vi "FlexMag - 23-03-2023.vi"() -> ()   [LabVIEW 2018] (continued)
            n3079 = In Range and Coerce(upper limit=3.0, x=w4898, lower limit=0.0 ("Elapsed Time (s)")) -> (In Range?=w4892:bool)  [unwired: 1 out]
            n3080 = Not(x=w4895) -> (.not. x?=w4894:bool)
            n3081 = local write "ch3 ch vbv timer"(w4894) -> ()
            n3082 = property on="chvbv3 timer tab" class="TabCtl (strict)"("Visible"=w4892) -> ()  [unwired: 2 in, 2 out]
          }
        }
        n3083 = feedback-in #98(w4536) -> ()
        n3084 = case shown="True" w4546 {
          tunnel: [TRUE FALSE] -> w4545
          tunnel: w4544 -> [_ w4913]
          frame False {
          }
          frame True {
            n3085 = call "Elapsed Time17"("Auto Reset"=w4913) -> ("Elapsed Time (s)"=w4918:dbl)  [unwired: 11 in, 7 out]
            n3086 = Greater?(x=w4918, y=3.0) -> (0:w4915:bool)
            n3087 = In Range and Coerce(upper limit=3.0, x=w4918, lower limit=0.0 ("Elapsed Time (s)")) -> (In Range?=w4912:bool)  [unwired: 1 out]
            n3088 = Not(x=w4915) -> (.not. x?=w4914:bool)
            n3089 = local write "ch1 ch vbv timer"(w4914) -> ()
            n3090 = property on="chvbv1 timer tab" class="TabCtl (strict)"("Visible"=w4912) -> ()  [unwired: 2 in, 2 out]
          }
        }
        n3091 = feedback-in #99(w4545) -> ()
        n3092 = case shown="True" w4564 {
          tunnel: [TRUE FALSE] -> w4563
          tunnel: w4562 -> [_ w4959]
          frame False {
          }
          frame True {
            n3093 = call "Elapsed Time12"("Auto Reset"=w4959) -> ("Elapsed Time (s)"=w4964:dbl)  [unwired: 11 in, 7 out]
            n3094 = Greater?(x=w4964, y=3.0) -> (0:w4961:bool)
            n3095 = In Range and Coerce(upper limit=3.0, x=w4964, lower limit=0.0 ("Elapsed Time (s)")) -> (In Range?=w4958:bool)  [unwired: 1 out]
            n3096 = Not(x=w4961) -> (.not. x?=w4960:bool)
            n3097 = local write "ch4 tp bv timer"(w4960) -> ()
            n3098 = property on="tpbv4 timer tab" class="TabCtl (strict)"("Visible"=w4958) -> ()  [unwired: 2 in, 2 out]
          }
        }
        n3099 = feedback-in #100(w4563) -> ()
        n3100 = case shown="True" w4565 {
          tunnel: [TRUE FALSE] -> w4566
          tunnel: w4567 -> [_ w4979]
          frame False {
          }
          frame True {
            n3101 = call "Elapsed Time10"("Auto Reset"=w4979) -> ("Elapsed Time (s)"=w4984:dbl)  [unwired: 11 in, 7 out]
            n3102 = Greater?(x=w4984, y=3.0) -> (0:w4981:bool)
            n3103 = In Range and Coerce(upper limit=3.0, x=w4984, lower limit=0.0 ("Elapsed Time (s)")) -> (In Range?=w4978:bool)  [unwired: 1 out]
            n3104 = Not(x=w4981) -> (.not. x?=w4980:bool)
            n3105 = local write "ch2 tp bv timer"(w4980) -> ()
            n3106 = property on="tpbv2 timer tab" class="TabCtl (strict)"("Visible"=w4978) -> ()  [unwired: 2 in, 2 out]
          }
        }
        n3107 = feedback-in #101(w4566) -> ()
        n3108 = case shown="True" w4559 {
          tunnel: [TRUE FALSE] -> w4560
          tunnel: w4561 -> [_ w4969]
          frame False {
          }
          frame True {
            n3109 = call "Elapsed Time11"("Auto Reset"=w4969) -> ("Elapsed Time (s)"=w4974:dbl)  [unwired: 11 in, 7 out]
            n3110 = Greater?(x=w4974, y=3.0) -> (0:w4971:bool)
            n3111 = In Range and Coerce(upper limit=3.0, x=w4974, lower limit=0.0 ("Elapsed Time (s)")) -> (In Range?=w4968:bool)  [unwired: 1 out]
            n3112 = Not(x=w4971) -> (.not. x?=w4970:bool)
            n3113 = local write "ch3 tp bv timer"(w4970) -> ()
            n3114 = property on="tpbv3 timer tab" class="TabCtl (strict)"("Visible"=w4968) -> ()  [unwired: 2 in, 2 out]
          }
        }
        n3115 = feedback-in #102(w4560) -> ()
        n3116 = case shown="True" w4588 {
          tunnel: [TRUE FALSE] -> w4587
          tunnel: w4586 -> [_ w5039]
          frame False {
          }
          frame True {
            n3117 = call "Elapsed Time4"("Auto Reset"=w5039) -> ("Elapsed Time (s)"=w5044:dbl)  [unwired: 11 in, 7 out]
            n3118 = Greater?(x=w5044, y=3.0) -> (0:w5041:bool)
            n3119 = In Range and Coerce(upper limit=3.0, x=w5044, lower limit=0.0 ("Elapsed Time (s)")) -> (In Range?=w5038:bool)  [unwired: 1 out]
            n3120 = Not(x=w5041) -> (.not. x?=w5040:bool)
            n3121 = property on="mp4 timer tab" class="TabCtl (strict)"("Visible"=w5038) -> ()  [unwired: 2 in, 2 out]
            n3122 = local write "ch4 mp timer"(w5040) -> ()
          }
        }
        n3123 = feedback-in #103(w4587) -> ()
        n3124 = case shown="True" w4570 {
          tunnel: [TRUE FALSE] -> w4569
          tunnel: w4568 -> [_ w4989]
          frame False {
          }
          frame True {
            n3125 = call "Elapsed Time9"("Auto Reset"=w4989) -> ("Elapsed Time (s)"=w4994:dbl)  [unwired: 11 in, 7 out]
            n3126 = Greater?(x=w4994, y=3.0) -> (0:w4991:bool)
            n3127 = In Range and Coerce(upper limit=3.0, x=w4994, lower limit=0.0 ("Elapsed Time (s)")) -> (In Range?=w4988:bool)  [unwired: 1 out]
            n3128 = Not(x=w4991) -> (.not. x?=w4990:bool)
            n3129 = local write "ch1 tp bv timer"(w4990) -> ()
            n3130 = property on="tpbv1 timer tab" class="TabCtl (strict)"("Visible"=w4988) -> ()  [unwired: 2 in, 2 out]
          }
        }
        n3131 = feedback-in #104(w4569) -> ()
        n3132 = case shown="True" w4589 {
          tunnel: [TRUE FALSE] -> w4590
          tunnel: w4591 -> [_ w5059]
          frame False {
          }
          frame True {
            n3133 = call "Elapsed Time2"("Auto Reset"=w5059) -> ("Elapsed Time (s)"=w5064:dbl)  [unwired: 11 in, 7 out]
            n3134 = Greater?(x=w5064, y=3.0) -> (0:w5061:bool)
            n3135 = In Range and Coerce(upper limit=3.0, x=w5064, lower limit=0.0 ("Elapsed Time (s)")) -> (In Range?=w5058:bool)  [unwired: 1 out]
            n3136 = Not(x=w5061) -> (.not. x?=w5060:bool)
            n3137 = property on="mp2 timer tab" class="TabCtl (strict)"("Visible"=w5058) -> ()  [unwired: 2 in, 2 out]
            n3138 = local write "ch2 mp timer"(w5060) -> ()
          }
        }
        n3139 = feedback-in #105(w4590) -> ()
        n3140 = case shown="True" w4583 {
          tunnel: [TRUE FALSE] -> w4584
          tunnel: w4585 -> [_ w5049]
          frame False {
          }
          frame True {
            n3141 = call "Elapsed Time3"("Auto Reset"=w5049) -> ("Elapsed Time (s)"=w5054:dbl)  [unwired: 11 in, 7 out]
            n3142 = Greater?(x=w5054, y=3.0) -> (0:w5051:bool)
            n3143 = In Range and Coerce(upper limit=3.0, x=w5054, lower limit=0.0 ("Elapsed Time (s)")) -> (In Range?=w5048:bool)  [unwired: 1 out]
            n3144 = Not(x=w5051) -> (.not. x?=w5050:bool)
            n3145 = property on="mp3 timer tab" class="TabCtl (strict)"("Visible"=w5048) -> ()  [unwired: 2 in, 2 out]
            n3146 = local write "ch3 mp timer"(w5050) -> ()
          }
        }
        n3147 = feedback-in #106(w4584) -> ()
        n3148 = case shown="True" w4594 {
          tunnel: [TRUE FALSE] -> w4593
          tunnel: w4592 -> [_ w5068]
          frame False {
          }
          frame True {
            n3149 = call "Elapsed Time"("Auto Reset"=w5068) -> ("Elapsed Time (s)"=w5074:dbl)  [unwired: 11 in, 7 out]
            n3150 = Greater?(x=w5074, y=3.0) -> (0:w5070:bool)
            n3151 = In Range and Coerce(upper limit=3.0, x=w5074, lower limit=0.0 ("Elapsed Time (s)")) -> (In Range?=w5071:bool)  [unwired: 1 out]
            n3152 = Not(x=w5070) -> (.not. x?=w5069:bool)
            n3153 = property on="mp1 timer tab" class="TabCtl (strict)"("Visible"=w5071) -> ()  [unwired: 2 in, 2 out]
            n3154 = local write "ch1 mp timer"(w5069) -> ()
          }
        }
        n3155 = feedback-in #107(w4593) -> ()
        n3156 = local read "ch4 pc gv timer"() -> (w4529:bool)
        n3157 = local read "ch2 pc gv timer"() -> (w4528:bool)
        n3158 = local read "ch3 pc gv timer"() -> (w4534:bool)
        n3159 = local read "ch1 pc gv timer"() -> (w4523:bool)
        n3160 = local read "ch4 pl vbv timer"() -> (w4577:bool)
        n3161 = local read "ch4 tp timer"() -> (w4481:bool)
        n3162 = local read "ch1 pl vbv timer"() -> (w4571:bool)
        n3163 = local read "ch2 pl vbv timer"() -> (w4576:bool)
        n3164 = local read "ch3 pl vbv timer"() -> (w4582:bool)
        n3165 = local read "ch2 tp timer"() -> (w4480:bool)
        n3166 = local read "ch3 tp timer"() -> (w4486:bool)
        n3167 = local read "ch1 tp timer"() -> (w4475:bool)
        n3168 = local read "ch4 cc timer"() -> (w4505:bool)
        n3169 = local read "ch2 cc timer"() -> (w4504:bool)
        n3170 = local read "ch3 cc timer"() -> (w4510:bool)
        n3171 = local read "ch1 cc timer"() -> (w4499:bool)
        n3172 = local read "ch4 tp timer"() -> (w4553:bool)
        n3173 = local read "ch2 tp timer"() -> (w4552:bool)
        n3174 = local read "ch3 tp timer"() -> (w4558:bool)
        n3175 = local read "ch1 tp timer"() -> (w4547:bool)
        n3176 = feedback #108() -> (w4483:bool)  [unwired: 1 in]
        n3177 = feedback #109() -> (w4478:bool)  [unwired: 1 in]
        n3178 = feedback #110() -> (w4484:bool)  [unwired: 1 in]
        n3179 = feedback #111() -> (w4477:bool)  [unwired: 1 in]
        n3180 = feedback #112() -> (w4507:bool)  [unwired: 1 in]
        n3181 = feedback #113() -> (w4531:bool)  [unwired: 1 in]
        n3182 = feedback #114() -> (w4502:bool)  [unwired: 1 in]
        n3183 = feedback #115() -> (w4508:bool)  [unwired: 1 in]
        n3184 = feedback #116() -> (w4526:bool)  [unwired: 1 in]
        n3185 = feedback #117() -> (w4532:bool)  [unwired: 1 in]
        n3186 = feedback #118() -> (w4501:bool)  [unwired: 1 in]
        n3187 = feedback #119() -> (w4525:bool)  [unwired: 1 in]
        n3188 = feedback #120() -> (w4555:bool)  [unwired: 1 in]
        n3189 = feedback #121() -> (w4550:bool)  [unwired: 1 in]
        n3190 = feedback #122() -> (w4556:bool)  [unwired: 1 in]
        n3191 = feedback #123() -> (w4549:bool)  [unwired: 1 in]
        n3192 = feedback #124() -> (w4579:bool)  [unwired: 1 in]
        n3193 = feedback #125() -> (w4573:bool)  [unwired: 1 in]
        n3194 = feedback #126() -> (w4574:bool)  [unwired: 1 in]
        n3195 = feedback #127() -> (w4580:bool)  [unwired: 1 in]
        n3196 = local read "ch4 trnsbp right timer"() -> (w4462:bool)
        n3197 = local read "ch2 trnsbp right timer"() -> (w4469:bool)
        n3198 = local read "ch3 trnsbp right timer"() -> (w4468:bool)
        n3199 = local read "ch2 trnsbp left timer"() -> (w4463:bool)
        n3200 = local read "ch3 trnsbp left timer"() -> (w4457:bool)
        n3201 = local read "ch1 trnsbp left timer"() -> (w4474:bool)
        n3202 = case shown="True" w4481 {
          tunnel: [TRUE FALSE] -> w4482
          tunnel: w4483 -> [_ w4687]
          frame False {
          }
          frame True {
            n3203 = call "Elapsed Time44"("Auto Reset"=w4687) -> ("Elapsed Time (s)"=w4692:dbl)  [unwired: 11 in, 7 out]
            n3204 = Greater?(x=w4692, y=3.0) -> (0:w4689:bool)
            n3205 = In Range and Coerce(upper limit=3.0, x=w4692, lower limit=0.0 ("Elapsed Time (s)")) -> (In Range?=w4686:bool)  [unwired: 1 out]
            n3206 = Not(x=w4689) -> (.not. x?=w4688:bool)
            n3207 = property on="tp4 timer tab" class="TabCtl (strict)"("Visible"=w4686) -> ()  [unwired: 2 in, 2 out]
            n3208 = local write "ch4 tp timer"(w4688) -> ()
          }
        }
        n3209 = feedback-in #108(w4482) -> ()
        n3210 = case shown="True" w4480 {
          tunnel: [TRUE FALSE] -> w4479
          tunnel: w4478 -> [_ w4707]
          frame False {
          }
          frame True {
            n3211 = call "Elapsed Time42"("Auto Reset"=w4707) -> ("Elapsed Time (s)"=w4712:dbl)  [unwired: 11 in, 7 out]
            n3212 = Greater?(x=w4712, y=3.0) -> (0:w4709:bool)
            n3213 = In Range and Coerce(upper limit=3.0, x=w4712, lower limit=0.0 ("Elapsed Time (s)")) -> (In Range?=w4706:bool)  [unwired: 1 out]
            n3214 = Not(x=w4709) -> (.not. x?=w4708:bool)
            n3215 = property on="tp2 timer tab" class="TabCtl (strict)"("Visible"=w4706) -> ()  [unwired: 2 in, 2 out]
            n3216 = local write "ch2 tp timer"(w4708) -> ()
          }
        }
        n3217 = feedback-in #109(w4479) -> ()
        n3218 = case shown="True" w4486 {
          tunnel: [TRUE FALSE] -> w4485
          tunnel: w4484 -> [_ w4697]
          frame False {
          }
          frame True {
            n3219 = call "Elapsed Time43"("Auto Reset"=w4697) -> ("Elapsed Time (s)"=w4702:dbl)  [unwired: 11 in, 7 out]
            n3220 = Greater?(x=w4702, y=3.0) -> (0:w4699:bool)
            n3221 = In Range and Coerce(upper limit=3.0, x=w4702, lower limit=0.0 ("Elapsed Time (s)")) -> (In Range?=w4696:bool)  [unwired: 1 out]
            n3222 = Not(x=w4699) -> (.not. x?=w4698:bool)
            n3223 = property on="tp3 timer tab" class="TabCtl (strict)"("Visible"=w4696) -> ()  [unwired: 2 in, 2 out]
            n3224 = local write "ch3 tp timer"(w4698) -> ()
          }
        }
        n3225 = feedback-in #110(w4485) -> ()
        n3226 = case shown="True" w4475 {
          tunnel: [TRUE FALSE] -> w4476
          tunnel: w4477 -> [_ w4717]
          frame False {
          }
          frame True {
            n3227 = call "Elapsed Time41"("Auto Reset"=w4717) -> ("Elapsed Time (s)"=w4722:dbl)  [unwired: 11 in, 7 out]
            n3228 = Greater?(x=w4722, y=3.0) -> (0:w4719:bool)
            n3229 = In Range and Coerce(upper limit=3.0, x=w4722, lower limit=0.0 ("Elapsed Time (s)")) -> (In Range?=w4716:bool)  [unwired: 1 out]
            n3230 = Not(x=w4719) -> (.not. x?=w4718:bool)
            n3231 = property on="tp1 timer tab" class="TabCtl (strict)"("Visible"=w4716) -> ()  [unwired: 2 in, 2 out]
            n3232 = local write "ch1 tp timer"(w4718) -> ()
          }
        }
        n3233 = feedback-in #111(w4476) -> ()
        n3234 = case shown="True" w4505 {
          tunnel: [TRUE FALSE] -> w4506
          tunnel: w4507 -> [_ w4767]
          frame False {
          }
          frame True {
            n3235 = call "Elapsed Time32"("Auto Reset"=w4767) -> ("Elapsed Time (s)"=w4772:dbl)  [unwired: 11 in, 7 out]
            n3236 = Greater?(x=w4772, y=3.0) -> (0:w4769:bool)
            n3237 = In Range and Coerce(upper limit=3.0, x=w4772, lower limit=0.0 ("Elapsed Time (s)")) -> (In Range?=w4766:bool)  [unwired: 1 out]
            n3238 = Not(x=w4769) -> (.not. x?=w4768:bool)
            n3239 = local write "ch4 cc timer"(w4768) -> ()
            n3240 = property on="cc4 timer tab" class="TabCtl (strict)"("Visible"=w4766) -> ()  [unwired: 2 in, 2 out]
          }
        }
        n3241 = feedback-in #112(w4506) -> ()
        n3242 = case shown="True" w4529 {
          tunnel: [TRUE FALSE] -> w4530
          tunnel: w4531 -> [_ w4846]
          frame False {
          }
          frame True {
            n3243 = call "Elapsed Time24"("Auto Reset"=w4846) -> ("Elapsed Time (s)"=w4851:dbl)  [unwired: 11 in, 7 out]
            n3244 = Greater?(x=w4851, y=3.0) -> (0:w4848:bool)
            n3245 = In Range and Coerce(upper limit=3.0, x=w4851, lower limit=0.0 ("Elapsed Time (s)")) -> ()  [unwired: 2 out]
            n3246 = Not(x=w4848) -> (.not. x?=w4847:bool)
            n3247 = local write "ch4 pc gv timer"(w4847) -> ()
          }
        }
        n3248 = feedback-in #113(w4530) -> ()
        n3249 = case shown="True" w4504 {
          tunnel: [TRUE FALSE] -> w4503
          tunnel: w4502 -> [_ w4787]
          frame False {
          }
          frame True {
            n3250 = call "Elapsed Time30"("Auto Reset"=w4787) -> ("Elapsed Time (s)"=w4792:dbl)  [unwired: 11 in, 7 out]
            n3251 = Greater?(x=w4792, y=3.0) -> (0:w4789:bool)
            n3252 = In Range and Coerce(upper limit=3.0, x=w4792, lower limit=0.0 ("Elapsed Time (s)")) -> (In Range?=w4786:bool)  [unwired: 1 out]
            n3253 = Not(x=w4789) -> (.not. x?=w4788:bool)
            n3254 = property on="cc2 timer tab" class="TabCtl (strict)"("Visible"=w4786) -> ()  [unwired: 2 in, 2 out]
            n3255 = local write "ch2 cc timer"(w4788) -> ()
          }
        }
        n3256 = feedback-in #114(w4503) -> ()
        n3257 = case shown="True" w4510 {
          tunnel: [TRUE FALSE] -> w4509
          tunnel: w4508 -> [_ w4777]
          frame False {
          }
          frame True {
            n3258 = call "Elapsed Time31"("Auto Reset"=w4777) -> ("Elapsed Time (s)"=w4782:dbl)  [unwired: 11 in, 7 out]
            n3259 = Greater?(x=w4782, y=3.0) -> (0:w4779:bool)
            n3260 = In Range and Coerce(upper limit=3.0, x=w4782, lower limit=0.0 ("Elapsed Time (s)")) -> (In Range?=w4776:bool)  [unwired: 1 out]
            n3261 = Not(x=w4779) -> (.not. x?=w4778:bool)
            n3262 = local write "ch3 cc timer"(w4778) -> ()
            n3263 = property on="cc3 timer tab" class="TabCtl (strict)"("Visible"=w4776) -> ()  [unwired: 2 in, 2 out]
          }
        }
        n3264 = feedback-in #115(w4509) -> ()
        n3265 = case shown="True" w4528 {
          tunnel: [TRUE FALSE] -> w4527
          tunnel: w4526 -> [_ w4864]
          frame False {
          }
          frame True {
            n3266 = call "Elapsed Time22"("Auto Reset"=w4864) -> ("Elapsed Time (s)"=w4869:dbl)  [unwired: 11 in, 7 out]
            n3267 = Greater?(x=w4869, y=3.0) -> (0:w4866:bool)
            n3268 = In Range and Coerce(upper limit=3.0, x=w4869, lower limit=0.0 ("Elapsed Time (s)")) -> ()  [unwired: 2 out]
            n3269 = Not(x=w4866) -> (.not. x?=w4865:bool)
            n3270 = local write "ch2 pc gv timer"(w4865) -> ()
          }
        }
        n3271 = feedback-in #116(w4527) -> ()
        n3272 = case shown="True" w4534 {
          tunnel: [TRUE FALSE] -> w4533
          tunnel: w4532 -> [_ w4855]
          frame False {
          }
          frame True {
            n3273 = call "Elapsed Time23"("Auto Reset"=w4855) -> ("Elapsed Time (s)"=w4860:dbl)  [unwired: 11 in, 7 out]
            n3274 = Greater?(x=w4860, y=3.0) -> (0:w4857:bool)
            n3275 = In Range and Coerce(upper limit=3.0, x=w4860, lower limit=0.0 ("Elapsed Time (s)")) -> ()  [unwired: 2 out]
            n3276 = Not(x=w4857) -> (.not. x?=w4856:bool)
            n3277 = local write "ch3 pc gv timer"(w4856) -> ()
          }
        }
        n3278 = feedback-in #117(w4533) -> ()
        n3279 = case shown="True" w4499 {
          tunnel: [TRUE FALSE] -> w4500
          tunnel: w4501 -> [_ w4797]
          frame False {
          }
          frame True {
            n3280 = call "Elapsed Time29"("Auto Reset"=w4797) -> ("Elapsed Time (s)"=w4802:dbl)  [unwired: 11 in, 7 out]
            n3281 = Greater?(x=w4802, y=3.0) -> (0:w4799:bool)
            n3282 = In Range and Coerce(upper limit=3.0, x=w4802, lower limit=0.0 ("Elapsed Time (s)")) -> (In Range?=w4796:bool)  [unwired: 1 out]
            n3283 = Not(x=w4799) -> (.not. x?=w4798:bool)
            n3284 = local write "ch1 cc timer"(w4798) -> ()
            n3285 = property on="cc1 timer tab" class="TabCtl (strict)"("Visible"=w4796) -> ()  [unwired: 2 in, 2 out]
          }
        }
        n3286 = feedback-in #118(w4500) -> ()
        n3287 = case shown="True" w4523 {
          tunnel: [TRUE FALSE] -> w4524
          tunnel: w4525 -> [_ w4873]
          frame False {
          }
          frame True {
            n3288 = call "Elapsed Time21"("Auto Reset"=w4873) -> ("Elapsed Time (s)"=w4878:dbl)  [unwired: 11 in, 7 out]
            n3289 = Greater?(x=w4878, y=3.0) -> (0:w4875:bool)
            n3290 = In Range and Coerce(upper limit=3.0, x=w4878, lower limit=0.0 ("Elapsed Time (s)")) -> ()  [unwired: 2 out]
            n3291 = Not(x=w4875) -> (.not. x?=w4874:bool)
            n3292 = local write "ch1 pc gv timer"(w4874) -> ()
          }
        }
        n3293 = feedback-in #119(w4524) -> ()
        n3294 = case shown="True" w4553 {
          tunnel: [TRUE FALSE] -> w4554
          tunnel: w4555 -> [_ w4922]
          frame False {
          }
          frame True {
            n3295 = call "Elapsed Time16"("Auto Reset"=w4922) -> ("Elapsed Time (s)"=w4927:dbl)  [unwired: 11 in, 7 out]
            n3296 = Greater?(x=w4927, y=3.0) -> (0:w4924:bool)
            n3297 = In Range and Coerce(upper limit=3.0, x=w4927, lower limit=0.0 ("Elapsed Time (s)")) -> ()  [unwired: 2 out]
            n3298 = Not(x=w4924) -> (.not. x?=w4923:bool)
            n3299 = local write "ch4 tp timer"(w4923) -> ()
          }
        }
        n3300 = feedback-in #120(w4554) -> ()
        n3301 = case shown="True" w4552 {
          tunnel: [TRUE FALSE] -> w4551
          tunnel: w4550 -> [_ w4940]
          frame False {
          }
          frame True {
            n3302 = call "Elapsed Time14"("Auto Reset"=w4940) -> ("Elapsed Time (s)"=w4945:dbl)  [unwired: 11 in, 7 out]
            n3303 = Greater?(x=w4945, y=3.0) -> (0:w4942:bool)
            n3304 = In Range and Coerce(upper limit=3.0, x=w4945, lower limit=0.0 ("Elapsed Time (s)")) -> ()  [unwired: 2 out]
            n3305 = Not(x=w4942) -> (.not. x?=w4941:bool)
            n3306 = local write "ch2 tp timer"(w4941) -> ()
          }
        }
        n3307 = feedback-in #121(w4551) -> ()
        n3308 = case shown="True" w4558 {
          tunnel: [TRUE FALSE] -> w4557
          tunnel: w4556 -> [_ w4931]
          frame False {
          }
          frame True {
            n3309 = call "Elapsed Time15"("Auto Reset"=w4931) -> ("Elapsed Time (s)"=w4936:dbl)  [unwired: 11 in, 7 out]
            n3310 = Greater?(x=w4936, y=3.0) -> (0:w4933:bool)
            n3311 = In Range and Coerce(upper limit=3.0, x=w4936, lower limit=0.0 ("Elapsed Time (s)")) -> ()  [unwired: 2 out]
            n3312 = Not(x=w4933) -> (.not. x?=w4932:bool)
            n3313 = local write "ch3 tp timer"(w4932) -> ()
          }
        }
        n3314 = feedback-in #122(w4557) -> ()
        n3315 = case shown="True" w4547 {
          tunnel: [TRUE FALSE] -> w4548
          tunnel: w4549 -> [_ w4949]
          frame False {
          }
          frame True {
            n3316 = call "Elapsed Time13"("Auto Reset"=w4949) -> ("Elapsed Time (s)"=w4954:dbl)  [unwired: 11 in, 7 out]
            n3317 = Greater?(x=w4954, y=3.0) -> (0:w4951:bool)
            n3318 = In Range and Coerce(upper limit=3.0, x=w4954, lower limit=0.0 ("Elapsed Time (s)")) -> ()  [unwired: 2 out]
            n3319 = Not(x=w4951) -> (.not. x?=w4950:bool)
            n3320 = local write "ch1 tp timer"(w4950) -> ()
          }
        }
        n3321 = feedback-in #123(w4548) -> ()
        n3322 = case shown="True" w4577 {
          tunnel: [TRUE FALSE] -> w4578
          tunnel: w4579 -> [_ w4999]
          frame False {
          }
          frame True {
            n3323 = call "Elapsed Time8"("Auto Reset"=w4999) -> ("Elapsed Time (s)"=w5004:dbl)  [unwired: 11 in, 7 out]
            n3324 = Greater?(x=w5004, y=3.0) -> (0:w5001:bool)
            n3325 = In Range and Coerce(upper limit=3.0, x=w5004, lower limit=0.0 ("Elapsed Time (s)")) -> (In Range?=w4998:bool)  [unwired: 1 out]
            n3326 = Not(x=w5001) -> (.not. x?=w5000:bool)
            n3327 = local write "ch4 pl vbv timer"(w5000) -> ()
            n3328 = property on="plvbv4 timer tab" class="TabCtl (strict)"("Visible"=w4998) -> ()  [unwired: 2 in, 2 out]
          }
        }
        n3329 = feedback-in #124(w4578) -> ()
        n3330 = case shown="True" w4571 {
          tunnel: [TRUE FALSE] -> w4572
          tunnel: w4573 -> [_ w5029]
          frame False {
          }
          frame True {
            n3331 = call "Elapsed Time5"("Auto Reset"=w5029) -> ("Elapsed Time (s)"=w5034:dbl)  [unwired: 11 in, 7 out]
            n3332 = Greater?(x=w5034, y=3.0) -> (0:w5031:bool)
            n3333 = In Range and Coerce(upper limit=3.0, x=w5034, lower limit=0.0 ("Elapsed Time (s)")) -> (In Range?=w5028:bool)  [unwired: 1 out]
            n3334 = Not(x=w5031) -> (.not. x?=w5030:bool)
            n3335 = local write "ch1 pl vbv timer"(w5030) -> ()
            n3336 = property on="plvbv1 timer tab" class="TabCtl (strict)"("Visible"=w5028) -> ()  [unwired: 2 in, 2 out]
          }
        }
        n3337 = feedback-in #125(w4572) -> ()
        n3338 = case shown="True" w4576 {
          tunnel: [TRUE FALSE] -> w4575
          tunnel: w4574 -> [_ w5019]
          frame False {
          }
          frame True {
            n3339 = call "Elapsed Time6"("Auto Reset"=w5019) -> ("Elapsed Time (s)"=w5024:dbl)  [unwired: 11 in, 7 out]
            n3340 = Greater?(x=w5024, y=3.0) -> (0:w5021:bool)
            n3341 = In Range and Coerce(upper limit=3.0, x=w5024, lower limit=0.0 ("Elapsed Time (s)")) -> (In Range?=w5018:bool)  [unwired: 1 out]
            n3342 = Not(x=w5021) -> (.not. x?=w5020:bool)
            n3343 = local write "ch2 pl vbv timer"(w5020) -> ()
            n3344 = property on="plvbv2 timer tab" class="TabCtl (strict)"("Visible"=w5018) -> ()  [unwired: 2 in, 2 out]
          }
        }
        n3345 = feedback-in #126(w4575) -> ()
        n3346 = case shown="True" w4582 {
          tunnel: [TRUE FALSE] -> w4581
          tunnel: w4580 -> [_ w5009]
          frame False {
          }
          frame True {
            n3347 = call "Elapsed Time7"("Auto Reset"=w5009) -> ("Elapsed Time (s)"=w5014:dbl)  [unwired: 11 in, 7 out]
            n3348 = Greater?(x=w5014, y=3.0) -> (0:w5011:bool)
            n3349 = In Range and Coerce(upper limit=3.0, x=w5014, lower limit=0.0 ("Elapsed Time (s)")) -> (In Range?=w5008:bool)  [unwired: 1 out]
            n3350 = Not(x=w5011) -> (.not. x?=w5010:bool)
            n3351 = local write "ch3 pl vbv timer"(w5010) -> ()
            n3352 = property on="plvbv3 timer tab" class="TabCtl (strict)"("Visible"=w5008) -> ()  [unwired: 2 in, 2 out]
          }
        }
        n3353 = feedback-in #127(w4581) -> ()
        n3354 = feedback #128() -> (w4460:bool)  [unwired: 1 in]
        n3355 = feedback #129() -> (w4459:bool)  [unwired: 1 in]
        n3356 = feedback #130() -> (w4466:bool)  [unwired: 1 in]
        n3357 = feedback #131() -> (w4471:bool)  [unwired: 1 in]
        n3358 = feedback #132() -> (w4465:bool)  [unwired: 1 in]
        n3359 = feedback #133() -> (w4472:bool)  [unwired: 1 in]
        n3360 = case shown="True" w4462 {
          tunnel: [TRUE FALSE] -> w4461
          tunnel: w4460 -> [_ w4627]
          frame False {
          }
          frame True {
            n3361 = call "Elapsed Time54"("Auto Reset"=w4627) -> ("Elapsed Time (s)"=w4632:dbl)  [unwired: 11 in, 7 out]
            n3362 = Greater?(x=w4632, y=3.0) -> (0:w4629:bool)
            n3363 = In Range and Coerce(upper limit=3.0, x=w4632, lower limit=0.0 ("Elapsed Time (s)")) -> (In Range?=w4626:bool)  [unwired: 1 out]
            n3364 = Not(x=w4629) -> (.not. x?=w4628:bool)
            n3365 = property on="ch4 trnsbp right timer tab" class="TabCtl (strict)"("Visible"=w4626) -> ()  [unwired: 2 in, 2 out]
            n3366 = local write "ch4 trnsbp right timer"(w4628) -> ()
          }
        }
        n3367 = feedback-in #128(w4461) -> ()
        n3368 = case shown="True" w4457 {
          tunnel: [TRUE FALSE] -> w4458
          tunnel: w4459 -> [_ w4637]
          frame False {
          }
          frame True {
            n3369 = call "Elapsed Time53"("Auto Reset"=w4637) -> ("Elapsed Time (s)"=w4642:dbl)  [unwired: 11 in, 7 out]
            n3370 = Greater?(x=w4642, y=3.0) -> (0:w4639:bool)
            n3371 = In Range and Coerce(upper limit=3.0, x=w4642, lower limit=0.0 ("Elapsed Time (s)")) -> (In Range?=w4636:bool)  [unwired: 1 out]
            n3372 = Not(x=w4639) -> (.not. x?=w4638:bool)
            n3373 = property on="ch3 trnsbp left timer tab" class="TabCtl (strict)"("Visible"=w4636) -> ()  [unwired: 2 in, 2 out]
            n3374 = local write "ch3 trnsbp left timer"(w4638) -> ()
          }
        }
        n3375 = feedback-in #129(w4458) -> ()
        n3376 = case shown="True" w4468 {
          tunnel: [TRUE FALSE] -> w4467
          tunnel: w4466 -> [_ w4647]
          frame False {
          }
          frame True {
            n3377 = call "Elapsed Time52"("Auto Reset"=w4647) -> ("Elapsed Time (s)"=w4652:dbl)  [unwired: 11 in, 7 out]
            n3378 = Greater?(x=w4652, y=3.0) -> (0:w4649:bool)
            n3379 = In Range and Coerce(upper limit=3.0, x=w4652, lower limit=0.0 ("Elapsed Time (s)")) -> (In Range?=w4646:bool)  [unwired: 1 out]
            n3380 = Not(x=w4649) -> (.not. x?=w4648:bool)
            n3381 = property on="ch3 trnsbp right timer tab" class="TabCtl (strict)"("Visible"=w4646) -> ()  [unwired: 2 in, 2 out]
            n3382 = local write "ch3 trnsbp right timer"(w4648) -> ()
          }
        }
        n3383 = feedback-in #130(w4467) -> ()
        n3384 = case shown="True" w4469 {
          tunnel: [TRUE FALSE] -> w4470
          tunnel: w4471 -> [_ w4667]
          frame False {
          }
          frame True {
            n3385 = call "Elapsed Time50"("Auto Reset"=w4667) -> ("Elapsed Time (s)"=w4672:dbl)  [unwired: 11 in, 7 out]
            n3386 = Greater?(x=w4672, y=3.0) -> (0:w4669:bool)
            n3387 = In Range and Coerce(upper limit=3.0, x=w4672, lower limit=0.0 ("Elapsed Time (s)")) -> (In Range?=w4666:bool)  [unwired: 1 out]
            n3388 = Not(x=w4669) -> (.not. x?=w4668:bool)
            n3389 = property on="ch2 trnsbp right timer tab" class="TabCtl (strict)"("Visible"=w4666) -> ()  [unwired: 2 in, 2 out]
            n3390 = local write "ch2 trnsbp right timer"(w4668) -> ()
          }
        }
        n3391 = feedback-in #131(w4470) -> ()
        n3392 = case shown="True" w4463 {
          tunnel: [TRUE FALSE] -> w4464
          tunnel: w4465 -> [_ w4657]
          frame False {
          }
          frame True {
            n3393 = call "Elapsed Time51"("Auto Reset"=w4657) -> ("Elapsed Time (s)"=w4662:dbl)  [unwired: 11 in, 7 out]
            n3394 = Greater?(x=w4662, y=3.0) -> (0:w4659:bool)
            n3395 = In Range and Coerce(upper limit=3.0, x=w4662, lower limit=0.0 ("Elapsed Time (s)")) -> (In Range?=w4656:bool)  [unwired: 1 out]
            n3396 = Not(x=w4659) -> (.not. x?=w4658:bool)
            n3397 = property on="ch2 trnsbp left timer tab" class="TabCtl (strict)"("Visible"=w4656) -> ()  [unwired: 2 in, 2 out]
            n3398 = local write "ch2 trnsbp left timer"(w4658) -> ()
          }
        }
        n3399 = feedback-in #132(w4464) -> ()
        n3400 = case shown="True" w4474 {
          tunnel: [TRUE FALSE] -> w4473
          tunnel: w4472 -> [_ w4677]
          frame False {
          }
          frame True {
            n3401 = call "Elapsed Time49"("Auto Reset"=w4677) -> ("Elapsed Time (s)"=w4682:dbl)  [unwired: 11 in, 7 out]
            n3402 = Greater?(x=w4682, y=3.0) -> (0:w4679:bool)
            n3403 = In Range and Coerce(upper limit=3.0, x=w4682, lower limit=0.0 ("Elapsed Time (s)")) -> (In Range?=w4676:bool)  [unwired: 1 out]
            n3404 = Not(x=w4679) -> (.not. x?=w4678:bool)
            n3405 = property on="ch1 trnsbp left timer tab" class="TabCtl (strict)"("Visible"=w4676) -> ()  [unwired: 2 in, 2 out]
            n3406 = local write "ch1 trnsbp left timer"(w4678) -> ()
          }
        }
        n3407 = feedback-in #133(w4473) -> ()
      }
      frame #6 {
        n3408 = local read "CH2_SRV1_Piston_Back_DI"() -> (w5106:bool)
        n3409 = local read "CH3_SRV1_Piston_Back_DI"() -> (w5110:bool)
        n3410 = local read "CH4_SRV1_Piston_Back_DI"() -> (w5107:bool)
        n3411 = local read "CH1_SRV1_Piston_Back_DI"() -> (w5111:bool)
        n3412 = local read "CH2_SRV1_Piston_For_DI"() -> (w5105:bool)
        n3413 = local read "CH3_SRV1_Piston_For_DI"() -> (w5109:bool)
        n3414 = local read "CH4_SRV1_Piston_For_DI"() -> (w5108:bool)
        n3415 = local read "CH2_PetCool_Down_DI"() -> (w5103:bool)
        n3416 = local read "CH3_PetCool_Down_DI"() -> (w5099:bool)
        n3417 = local read "CH4_PetCool_Down_DI"() -> (w5102:bool)
        n3418 = local read "CH1_SRV1_Piston_For_DI"() -> (w5112:bool)
        n3419 = local read "CH1_PetCool_Down_DI"() -> (w5098:bool)
        n3420 = local read "CH2_Cst_Fix_Down_DI"() -> (w5090:bool)
        n3421 = local read "CH3_Cst_Fix_Down_DI"() -> (w5094:bool)
        n3422 = local read "CH4_Cst_Fix_Down_DI"() -> (w5091:bool)
        n3423 = local read "CH1_Cst_Fix_Down_DI"() -> (w5095:bool)
        n3424 = local read "CH2_PetCool_Up_DI"() -> (w5104:bool)
        n3425 = local read "CH3_PetCool_Up_DI"() -> (w5100:bool)
        n3426 = local read "CH4_PetCool_Up_DI"() -> (w5101:bool)
        n3427 = local read "CH1_PetCool_Up_DI"() -> (w5097:bool)
        n3428 = local read "CH2_Cst_Fix_Up_DI"() -> (w5089:bool)
        n3429 = local read "CH3_Cst_Fix_Up_DI"() -> (w5093:bool)
        n3430 = local read "CH4_Cst_Fix_Up_DI"() -> (w5092:bool)
        n3431 = local read "CH1_Cst_Fix_Up_DI"() -> (w5096:bool)
        n3432 = local read "CH1_CH_ATM_DI"() -> (w5152:bool)
        n3433 = local read "CH2_CH_ATM_DI"() -> (w5151:bool)
        n3434 = local read "CH3_CH_ATM_DI"() -> (w5147:bool)
        n3435 = local read "CH1_PL_ATM_DI"() -> (w5153:bool)
        n3436 = local read "CH4_CH_ATM_DI"() -> (w5148:bool)
        n3437 = local read "CH2_PL_ATM_DI"() -> (w5150:bool)
        n3438 = local read "CH3_PL_ATM_DI"() -> (w5146:bool)
        n3439 = local read "CH4_PL_ATM_DI"() -> (w5149:bool)
        n3440 = local read "Warning Message"() -> (w5122:string)
        n3441 = local read "System Status"() -> (w5113:string)
        n3442 = case shown="True" w5104 {
          tunnel: w5103 -> [w5210 w5214]
          tunnel: [w5209 w5213] -> w5083
          frame False {
            n3443 = case shown="True" w5210 {
              tunnel: ["-----" ("x") "DOWN" ("x")] -> w5209
              frame False {
              }
              frame True {
              }
            }
          }
          frame True {
            n3444 = case shown="False" w5214 {
              tunnel: ["UP" ("x") "-----" ("x")] -> w5213
              frame False {
              }
              frame True {
              }
            }
          }
        }
        "ch2_petcool_status" <- w5083
        n3445 = case shown="True" w5100 {
          tunnel: w5099 -> [w5218 w5222]
          tunnel: [w5217 w5221] -> w5082
          frame False {
            n3446 = case shown="True" w5218 {
              tunnel: ["-----" ("x") "DOWN" ("x")] -> w5217
              frame False {
              }
              frame True {
              }
            }
          }
          frame True {
            n3447 = case shown="False" w5222 {
              tunnel: ["UP" ("x") "-----" ("x")] -> w5221
              frame False {
              }
              frame True {
              }
            }
          }
        }
        "ch3_petcool_status" <- w5082
        n3448 = case shown="True" w5101 {
          tunnel: w5102 -> [w5202 w5206]
          tunnel: [w5201 w5205] -> w5081
          frame False {
            n3449 = case shown="True" w5202 {
              tunnel: ["-----" ("x") "DOWN" ("x")] -> w5201
              frame False {
              }
              frame True {
              }
            }
          }
          frame True {
            n3450 = case shown="False" w5206 {
              tunnel: ["UP" ("x") "-----" ("x")] -> w5205
              frame False {
              }
              frame True {
              }
            }
          }
        }
        "ch4_petcool_status" <- w5081
        n3451 = case shown="False" w5089 {
          tunnel: w5090 -> [w5178 w5182]
          tunnel: [w5177 w5181] -> w5079
          frame False {
            n3452 = case shown="True" w5178 {
              tunnel: ["-----" ("x") "DOWN" ("x")] -> w5177
              frame False {
              }
              frame True {
              }
            }
          }
          frame True {
            n3453 = case shown="False" w5182 {
              tunnel: ["UP" ("x") "-----" ("x")] -> w5181
              frame False {
              }
              frame True {
              }
            }
          }
        }
        "ch2_cst_fix_status" <- w5079
        n3454 = case shown="False" w5093 {
          tunnel: w5094 -> [w5186 w5190]
          tunnel: [w5185 w5189] -> w5078
          frame False {
            n3455 = case shown="True" w5186 {
              tunnel: ["-----" ("x") "DOWN" ("x")] -> w5185
              frame False {
              }
              frame True {
              }
            }
          }
          frame True {
            n3456 = case shown="False" w5190 {
              tunnel: ["UP" ("x") "-----" ("x")] -> w5189
              frame False {
              }
              frame True {
              }
            }
          }
        }
        "ch3_cst_fix_status" <- w5078
        n3457 = case shown="False" w5092 {
          tunnel: w5091 -> [w5170 w5174]
          tunnel: [w5169 w5173] -> w5077
          frame False {
            n3458 = case shown="True" w5170 {
              tunnel: ["-----" ("x") "DOWN" ("x")] -> w5169
              frame False {
              }
              frame True {
              }
            }
          }
          frame True {
            n3459 = case shown="False" w5174 {
              tunnel: ["UP" ("x") "-----" ("x")] -> w5173
              frame False {
              }
              frame True {
              }
            }
          }
        }
        "ch4_cst_fix_status" <- w5077
        n3460 = case shown="False" w5105 {
          tunnel: w5106 -> [w5242 w5246]
          tunnel: [w5241 w5245] -> w5087
          frame False {
            n3461 = case shown="True" w5242 {
              tunnel: ["-----" ("x") "DECOUPLED" ("x")] -> w5241
              frame False {
              }
              frame True {
              }
            }
          }
          frame True {
            n3462 = case shown="False" w5246 {
              tunnel: ["COUPLED" ("x") "-----" ("x")] -> w5245
              frame False {
              }
              frame True {
              }
            }
          }
        }
        "ch2_srv_piston_status" <- w5087
        n3463 = case shown="False" w5109 {
          tunnel: w5110 -> [w5250 w5254]
          tunnel: [w5249 w5253] -> w5086
          frame False {
            n3464 = case shown="True" w5250 {
              tunnel: ["-----" ("x") "DECOUPLED" ("x")] -> w5249
              frame False {
              }
              frame True {
              }
            }
          }
          frame True {
            n3465 = case shown="False" w5254 {
              tunnel: ["COUPLED" ("x") "-----" ("x")] -> w5253
              frame False {
              }
              frame True {
              }
            }
          }
        }
        "ch3_srv_piston_status" <- w5086
        n3466 = case shown="False" w5108 {
          tunnel: w5107 -> [w5234 w5238]
          tunnel: [w5233 w5237] -> w5085
          frame False {
            n3467 = case shown="True" w5234 {
              tunnel: ["-----" ("x") "DECOUPLED" ("x")] -> w5233
              frame False {
              }
              frame True {
              }
            }
          }
          frame True {
            n3468 = case shown="False" w5238 {
              tunnel: ["COUPLED" ("x") "-----" ("x")] -> w5237
              frame False {
              }
              frame True {
              }
            }
          }
        }
        "ch4_srv_piston_status" <- w5085
        n3469 = case shown="True" w5097 {
          tunnel: w5098 -> [w5226 w5230]
          tunnel: [w5225 w5229] -> w5084
          frame False {
            n3470 = case shown="True" w5226 {
              tunnel: ["-----" ("x") "DOWN" ("x")] -> w5225
              frame False {
              }
              frame True {
              }
            }
          }
          frame True {
            n3471 = case shown="False" w5230 {
              tunnel: ["UP" ("x") "-----" ("x")] -> w5229
              frame False {
              }
              frame True {
              }
            }
          }
        }
        "ch1_petcool_status" <- w5084
        n3472 = case shown="False" w5096 {
          tunnel: w5095 -> [w5194 w5198]
          tunnel: [w5193 w5197] -> w5080
          frame False {
            n3473 = case shown="True" w5194 {
              tunnel: ["-----" ("x") "DOWN" ("x")] -> w5193
              frame False {
              }
              frame True {
              }
            }
          }
          frame True {
            n3474 = case shown="False" w5198 {
              tunnel: ["UP" ("x") "-----" ("x")] -> w5197
              frame False {
              }
              frame True {
              }
            }
          }
        }
        "ch1_cst_fix_status" <- w5080
        n3475 = case shown="False" w5112 {
          tunnel: w5111 -> [w5258 w5262]
          tunnel: [w5257 w5261] -> w5088
          frame False {
            n3476 = case shown="True" w5258 {
              tunnel: ["-----" ("x") "DECOUPLED" ("x")] -> w5257
              frame False {
              }
              frame True {
              }
            }
          }
          frame True {
            n3477 = case shown="True" w5262 {
              tunnel: ["COUPLED" ("x") "-----" ("x")] -> w5261
              frame False {
              }
              frame True {
              }
            }
          }
        }
        "ch1_srv_piston_status" <- w5088
        n3478 = case shown="True" w5153 {
          frame False {
          }
          frame True {
            n3479 = local write "CH1_PL_VBV_DO"(FALSE) -> ()
          }
        }
        n3480 = case shown="True" w5150 {
          frame False {
          }
          frame True {
            n3481 = local write "CH2_PL_VBV_DO"(FALSE) -> ()
          }
        }
        n3482 = case shown="True" w5152 {
          frame False {
          }
          frame True {
            n3483 = local write "CH1_CH_VBV_DO"(FALSE) -> ()
          }
        }
        n3484 = case shown="True" w5151 {
          frame False {
          }
          frame True {
            n3485 = local write "CH2_CH_VBV_DO"(FALSE) -> ()
          }
        }
        n3486 = case shown="True" w5146 {
          frame False {
          }
          frame True {
            n3487 = local write "CH3_PL_VBV_DO"(FALSE) -> ()
          }
        }
        n3488 = case shown="True" w5149 {
          frame False {
          }
          frame True {
            n3489 = local write "CH4_PL_VBV_DO"(FALSE) -> ()
          }
        }
        n3490 = case shown="True" w5147 {
          frame False {
          }
          frame True {
            n3491 = local write "CH3_CH_VBV_DO"(FALSE) -> ()
          }
        }
        n3492 = case shown="True" w5148 {
          frame False {
          }
          frame True {
            n3493 = local write "CH4_CH_VBV_DO"(FALSE) -> ()
          }
        }
        n3494 = feedback #134() -> (w5116:string)  [unwired: 1 in]
        n3495 = feedback-in #134(w5113) -> ()
        n3496 = feedback-in #135(w5122) -> ()
        n3497 = feedback #135() -> (w5124:string)  [unwired: 1 in]
        n3498 = Not Equal?(x="", y=w5113) -> (x != y?=w5114:bool)
        n3499 = Not Equal?(x=w5113, y=w5116) -> (x != y?=w5118:bool)
        n3500 = Not Equal?(x="", y=w5122) -> (x != y?=w5120:bool)
        n3501 = Not Equal?(x=w5122, y=w5124) -> (x != y?=w5119:bool)
        n3502 = And(x=w5114, y=w5118) -> (x .and. y?=w5115:bool)
        n3503 = And(x=w5120, y=w5119) -> (x .and. y?=w5123:bool)
        n3504 = Boolean Array To Number(Boolean array=w5167) -> (number=w5168:u32)
        n3505 = case shown="True" w5123 {
          tunnel: w5122 -> [_ w5275]
          frame False {
          }
          frame True {
            n3506 = Get Date/Time String(want seconds? (F)=TRUE) -> (date string=w5282:string, time string=w5279:string)  [unwired: 2 in]
            n3507 = local read "Total Warning"() -> (w5276:string)
            n3508 = call <vilib>:"Space Constant.vi"() -> ("String"=w5274:string)
            n3509 = Concatenate Strings(w5276, "\r\n", w5282, "-" ("string"), w5279, w5274, w5275) -> (→"Total Warning":string)
          }
        }
        n3510 = case shown="True" w5115 {
          tunnel: w5113 -> [_ w5266]
          frame False {
          }
          frame True {
            n3511 = local read "Total Status"() -> (w5267:string)
            n3512 = Get Date/Time String(want seconds? (F)=TRUE) -> (date string=w5269:string, time string=w5272:string)  [unwired: 2 in]
            n3513 = call <vilib>:"Space Constant.vi"() -> ("String"=w5265:string)
            n3514 = Concatenate Strings(w5267, "\r\n", w5269, "-" ("string"), w5272, w5265, w5266) -> (→"Total Status":string)
          }
        }
        n3515 = Boolean Array To Number(Boolean array=w5158) -> (number=w5159:u32)
        n3516 = Mantissa & Exponent(0:w5168) -> (2:w5154:dbl)  [unwired: 1 out]
        n3517 = Mantissa & Exponent(0:w5159) -> (2:w5155:dbl)  [unwired: 1 out]
        n3518 = Equal To 0?(x=w5155) -> (x = 0?=w5156:bool)
        n3519 = case shown="False" w5156 {
          tunnel: [w5317 w5320] -> w5157
          tunnel: w5155 -> [w5316 w5319]
          tunnel: w5154 -> [_ w5318]
          frame False {
            n3520 = Add(x=w5316, y=31.0) -> (x+y=w5317:dbl)
          }
          frame True {
            n3521 = Add(x=w5319, y=w5318) -> (x+y=w5320:dbl)
          }
        }
        n3522 = local read "WFC DI"() -> (w5143:bool)
        n3523 = local read "CH1 I/O Loading"() -> (w5140:bool)
        n3524 = local read "CH2 I/O Loading"() -> (w5139:bool)
        n3525 = local read "CH3 I/O Loading"() -> (w5137:bool)
        n3526 = local read "CH4 I/O Loading"() -> (w5138:bool)
        n3527 = feedback #136() -> (w5145:bool)  [unwired: 1 in]
        n3528 = local read "tp3 start safety"() -> (w5131:bool)
        n3529 = local read "tp4 start safety"() -> (w5132:bool)
        n3530 = local read "tp1 start safety"() -> (w5136:bool)
        n3531 = local read "tp2 start safety"() -> (w5134:bool)
        n3532 = case shown="20" w5157 {
          tunnel: ["" ("Description") "Chamber 4 Mechanical Pump" ("Description") "Chamber 3 Mechanical Pump" ("Description") "Chamber 2 Mechanical Pump" ("Description") "Chamber 1 Mechanical Pump" ("Description") "Chamber 4 Pipeline Vacuum Brake Valve" ("Description") "Chamber 3 Pipeline Vacuum Brake Valve" ("Description") "Chamber 2 Pipeline Vacuum Brake Valve" ("Description") "Chamber 1 Pipeline Vacuum Brake Valve" ("Description") "Chamber 4 Pipeline Pirani Gauge" ("Description") "Chamber 3 Pipeline Pirani Gauge" ("Description") "Chamber 2 Pipeline Pirani Gauge" ("Description") "Chamber 1 Pipeline Pirani Gauge" ("Description") "Chamber 4 Pipeline Atmospheric Switch" ("Description") "Chamber 3 Pipeline Atmospheric Switch" ("Description") "Chamber 2 Pipeline Atmospheric Switch" ("Description") "Chamber 1 Pipeline Atmospheric Switch" ("Description") "Chamber 4 Turbo Pump Block Valve" ("Description") "Chamber 3 Turbo Pump Block Valve" ("Description") "Chamber 2 Turbo Pump Block Valve" ("Description") "Chamber 1 Turbo Pump Block Valve" ("Description") "Chamber 4 Turbo Pump" ("Description") "Chamber 3 Turbo Pump" ("Description") "Chamber 2 Turbo Pump" ("Description") "Chamber 1 Turbo Pump" ("Description") "Chamber 4 Chamber Vacuum Brake Valve" ("Description") "Chamber 3 Chamber Vacuum Brake Valve" ("Description") "Chamber 2 Chamber Vacuum Brake Valve" ("Description") "Chamber 1 Chamber Vacuum Brake Valve" ("Description") "Chamber 4 Pressure Control Valve" ("Description") "Chamber 3 Pressure Control Valve" ("Description") "Chamber 2 Pressure Control Valve" ("Description") "Chamber 1 Pressure Control Valve" ("Description") "Chamber 4 Chamber Pirani Gauge" ("Description") "Chamber 3 Chamber Pirani Gauge" ("Description") "Chamber 2 Chamber Pirani Gauge" ("Description") "Chamber 1 Chamber Pirani Gauge" ("Description") "Chamber 4 Cold Cathode Gauge" ("Description") "Chamber 3 Cold Cathode Gauge" ("Description") "Chamber 2 Cold Cathode Gauge" ("Description") "Chamber 1 Cold Cathode Gauge" ("Description") "Chamber 4 Baratron Gauge Block Valve" ("Description") "Chamber 3 Baratron Gauge Block Valve" ("Description") "Chamber 2 Baratron Gauge Block Valve" ("Description") "Chamber 1 Baratron Gauge Block Valve" ("Description") "Chamber 4 Baratron Gauge" ("Description") "Chamber 3 Baratron Gauge" ("Description") "Chamber 2 Baratron Gauge" ("Description") "Chamber 1 Baratron Gauge" ("Description") "Chamber 4 Chamber Atmospheric Switch" ("Description") "Chamber 3 Chamber Atmospheric Switch" ("Description") "Chamber 2 Chamber Atmospheric Switch" ("Description") "Chamber 1 Chamber Atmospheric Switch" ("Description") "CH4-CH3 Transfer Gate Valve" ("Description") "CH3-CH2 Transfer Gate Valve" ("Description") "CH2-CH1 Transfer Gate Valve" ("Description") "Transfer Gate  Bypass Valve" ("Description") "Transfer Gate  Bypass Valve" ("Description") "Transfer Gate  Bypass Valve" ("Description") "Transfer Gate  Bypass Valve" ("Description") "Transfer Gate  Bypass Valve" ("Description") "Transfer Gate  Bypass Valve" ("Description")] -> w5164
          tunnel: ["" ("Description") "CH4 MP" ("Description") "CH3 MP" ("Description") "CH2 MP" ("Description") "CH1 MP" ("Description") "CH4 PL VBV" ("Description") "CH3 PL VBV" ("Description") "CH2 PL VBV" ("Description") "CH1 PL VBV" ("Description") "CH4 PL PG" ("Description") "CH3 PL PG" ("Description") "CH2 PL PG" ("Description") "CH1 PL PG" ("Description") "CH4 PL ATM" ("Description") "CH3 PL ATM" ("Description") "CH2 PL ATM" ("Description") "CH1 PL ATM" ("Description") "CH4 TP BV" ("Description") "CH3 TP BV" ("Description") "CH2 TP BV" ("Description") "CH1 TP BV" ("Description") "CH4 TP" ("Description") "CH3 TP" ("Description") "CH2 TP" ("Description") "CH1 TP" ("Description") "CH4 CH VBV" ("Description") "CH3 CH VBV" ("Description") "CH2 CH VBV" ("Description") "CH1 CH VBV" ("Description") "CH4 PC GV" ("Description") "CH3 PC GV" ("Description") "CH2 PC GV" ("Description") "CH1 PC GV" ("Description") "CH4 CH PG" ("Description") "CH3 CH PG" ("Description") "CH2 CH PG" ("Description") "CH1 CH PG" ("Description") "CH4 CC" ("Description") "CH3 CC" ("Description") "CH2 CC" ("Description") "CH1 CC" ("Description") "CH4 BG BV" ("Description") "CH3 BG BV" ("Description") "CH2 BG BV" ("Description") "CH1 BG BV" ("Description") "CH4 BG" ("Description") "CH3 BG" ("Description") "CH2 BG" ("Description") "CH1 BG" ("Description") "CH4 CH ATM" ("Description") "CH3 CH ATM" ("Description") "CH2 CH ATM" ("Description") "CH1 CH ATM" ("Description") "TRNS GV" ("Description") "TRNS GV" ("Description") "TRNS GV" ("Description") "TRNS GV BP" ("Description") "TRNS GV BP" ("Description") "TRNS GV BP" ("Description") "TRNS GV BP" ("Description") "TRNS GV BP" ("Description") "TRNS GV BP" ("Description")] -> w5163
          tunnel: [cluster{"x":i16, "y":i16} {"x"=0, "y"=0} ("origin") cluster{"x":i16, "y":i16} {"x"=220, "y"=76} ("origin") cluster{"x":i16, "y":i16} {"x"=544, "y"=76} ("origin") cluster{"x":i16, "y":i16} {"x"=870, "y"=76} ("origin") cluster{"x":i16, "y":i16} {"x"=1200, "y"=76} ("origin") cluster{"x":i16, "y":i16} {"x"=10, "y"=120} ("origin") cluster{"x":i16, "y":i16} {"x"=280, "y"=120} ("origin") cluster{"x":i16, "y":i16} {"x"=630, "y"=120} ("origin") cluster{"x":i16, "y":i16} {"x"=940, "y"=120} ("origin") cluster{"x":i16, "y":i16} {"x"=210, "y"=120} ("origin") cluster{"x":i16, "y":i16} {"x"=540, "y"=120} ("origin") cluster{"x":i16, "y":i16} {"x"=870, "y"=120} ("origin") cluster{"x":i16, "y":i16} {"x"=1180, "y"=120} ("origin") cluster{"x":i16, "y":i16} {"x"=230, "y"=240} ("origin") cluster{"x":i16, "y":i16} {"x"=550, "y"=240} ("origin") cluster{"x":i16, "y":i16} {"x"=880, "y"=240} ("origin") cluster{"x":i16, "y":i16} {"x"=1200, "y"=240} ("origin") cluster{"x":i16, "y":i16} {"x"=210, "y"=340} ("origin") cluster{"x":i16, "y":i16} {"x"=540, "y"=340} ("origin") cluster{"x":i16, "y":i16} {"x"=870, "y"=340} ("origin") cluster{"x":i16, "y":i16} {"x"=1200, "y"=340} ("origin") cluster{"x":i16, "y":i16} {"x"=220, "y"=400} ("origin") cluster{"x":i16, "y":i16} {"x"=550, "y"=400} ("origin") cluster{"x":i16, "y":i16} {"x"=880, "y"=400} ("origin") cluster{"x":i16, "y":i16} {"x"=1200, "y"=400} ("origin") cluster{"x":i16, "y":i16} {"x"=10, "y"=370} ("origin") cluster{"x":i16, "y":i16} {"x"=360, "y"=370} ("origin") cluster{"x":i16, "y":i16} {"x"=680, "y"=370} ("origin") cluster{"x":i16, "y":i16} {"x"=1000, "y"=370} ("origin") cluster{"x":i16, "y":i16} {"x"=240, "y"=420} ("origin") cluster{"x":i16, "y":i16} {"x"=550, "y"=420} ("origin") cluster{"x":i16, "y":i16} {"x"=870, "y"=420} ("origin") cluster{"x":i16, "y":i16} {"x"=1200, "y"=420} ("origin") cluster{"x":i16, "y":i16} {"x"=10, "y"=780} ("origin") cluster{"x":i16, "y":i16} {"x"=350, "y"=780} ("origin") cluster{"x":i16, "y":i16} {"x"=700, "y"=780} ("origin") cluster{"x":i16, "y":i16} {"x"=1000, "y"=780} ("origin") cluster{"x":i16, "y":i16} {"x"=60, "y"=790} ("origin") cluster{"x":i16, "y":i16} {"x"=400, "y"=790} ("origin") cluster{"x":i16, "y":i16} {"x"=750, "y"=790} ("origin") cluster{"x":i16, "y":i16} {"x"=1050, "y"=790} ("origin") cluster{"x":i16, "y":i16} {"x"=250, "y"=770} ("origin") cluster{"x":i16, "y":i16} {"x"=580, "y"=770} ("origin") cluster{"x":i16, "y":i16} {"x"=910, "y"=770} ("origin") cluster{"x":i16, "y":i16} {"x"=1196, "y"=770} ("origin") cluster{"x":i16, "y":i16} {"x"=250, "y"=770} ("origin") cluster{"x":i16, "y":i16} {"x"=580, "y"=770} ("origin") cluster{"x":i16, "y":i16} {"x"=910, "y"=770} ("origin") cluster{"x":i16, "y":i16} {"x"=1196, "y"=770} ("origin") cluster{"x":i16, "y":i16} {"x"=250, "y"=770} ("origin") cluster{"x":i16, "y":i16} {"x"=580, "y"=770} ("origin") cluster{"x":i16, "y":i16} {"x"=910, "y"=770} ("origin") cluster{"x":i16, "y":i16} {"x"=1196, "y"=770} ("origin") cluster{"x":i16, "y":i16} {"x"=300, "y"=696} ("origin") cluster{"x":i16, "y":i16} {"x"=620, "y"=696} ("origin") cluster{"x":i16, "y":i16} {"x"=950, "y"=696} ("origin") cluster{"x":i16, "y":i16} {"x"=950, "y"=430} ("origin") cluster{"x":i16, "y":i16} {"x"=900, "y"=430} ("origin") cluster{"x":i16, "y":i16} {"x"=590, "y"=430} ("origin") cluster{"x":i16, "y":i16} {"x"=570, "y"=430} ("origin") cluster{"x":i16, "y":i16} {"x"=280, "y"=430} ("origin") cluster{"x":i16, "y":i16} {"x"=240, "y"=430} ("origin")] -> w5162
          frame 0, Default {
          }
          frame 1 {
          }
          frame 2 {
          }
          frame 3 {
          }
          frame 4 {
          }
          frame 5 {
          }
          frame 6 {
          }
          frame 7 {
          }
          frame 8 {
          }
          frame 9 {
          }
          frame 10 {
          }
          frame 11 {
          }
          frame 12 {
          }
          frame 13 {
          }
          frame 14 {
          }
          frame 15 {
          }
          frame 16 {
          }
          frame 17 {
          }
          frame 18 {
          }
          frame 19 {
          }
          frame 20 {
          }
          frame 21 {
          }
          frame 22 {
          }
          frame 23 {
          }
          frame 24 {
          }
          frame 25 {
          }
          frame 26 {
          }
          frame 27 {
          }
          frame 28 {
          }
          frame 29 {
          }
          frame 30 {
          }
          frame 31 {
          }
          frame 32 {
          }
          frame 33 {
          }
          frame 34 {
          }
          frame 35 {
          }
          frame 36 {
          }
          frame 37 {
          }
          frame 38 {
          }
          frame 39 {
          }
          frame 40 {
          }
          frame 41 {
          }
          frame 42 {
          }
          frame 43 {
          }
          frame 44 {
          }
          frame 45 {
          }
          frame 46 {
          }
          frame 47 {
          }
          frame 48 {
          }
          frame 49 {
          }
          frame 50 {
          }
          frame 51 {
          }
          frame 52 {
          }
          frame 53 {
          }
          frame 54 {
          }
          frame 55 {
          }
          frame 56 {
          }
          frame 57 {
          }
          frame 58 {
          }
          frame 59 {
          }
          frame 60 {
          }
          frame 61 {
          }
        }
        n3533 = case shown="False" w5143 {
          tunnel: [FALSE TRUE] -> w5144
          tunnel: w5145 -> [w5299 _]
          tunnel: [w5300 FALSE] -> w5142
          frame False {
            n3534 = call "Elapsed Time146"("Reset"=w5299) -> ("Elapsed Time (s)"=w5302:dbl)  [unwired: 11 in, 7 out]
            n3535 = Greater Or Equal?(x=w5302, y=5.0) -> (x >= y?=w5300:bool)
          }
          frame True {
          }
        }
        n3536 = feedback-in #136(w5144) -> ()
        n3537 = local read "CH1_CC_DI"() -> (w5128:bool)
        n3538 = local read "CH2_CC_DI"() -> (w5127:bool)
        n3539 = local read "CH3_CC_DI"() -> (w5126:bool)